vi "HFRR ADV v043.vi"() -> ()   [LabVIEW 2025] (continued)
  # "Calibration completed successfully. The measured stroke length is within the acceptable tolerance range of the factory calibration value."
  # "Calibration failed. The measured stroke length differs from the factory calibration value by more than 20%. Please perform the calibration again."
  # "Step 1 — Ball Holder"
  # "Remove the ball holder by loosening and removing the center screw for Friction calibration."
  # "Step 2 — Disc Holder"
  # "Remove the disc holder by loosening and removing the opposing screws. Clean any fluid present in the disc holder."
  # "Step 3 — Calibration Head"
  # "Place the calibration holder in position and securely tighten the center screw."
  # "Step 4 — Calibration Holder"
  # "Place the calibration holder in position and tighten the two securing screws"
  # "Step 5 — Tare (Spring at Free Length)"
  # "Ensure the spring is at its contact (compressed) length — the micrometer head is in contact. Click Tare Sensor to zero the friction force baseline."
  # "Step 6 — Measure Friction Force"
  # "Run the Actual Test to measure Friction Force."
  # "Calibration in Progress"
  # "Step 7 — CALIBRATION RESULT"
  # "Calibration completed successfully. The measured friction force is within the acceptable tolerance range of the factory calibration value."
  # "Calibration failed. The measured friction force differs from the factory calibration value . Please perform the calibration again."
  # "Spring Constant: k = 1.000 N/mm\nSpring force |F| = k Ч d"
  # "Calibrates the sample/bath temperature sensor. \nUsed for test specimen and lubricant temperature measurement."
  # "Calibrates the ambient air temperature sensor. \nUsed for environmental chamber monitoring."
  # "Set B\n60 °C\nHigh-point calibration"
  # "Set A\n0 °C\nIce-point calibration"
  # "Set B\n60 °C\nHigh-point calibration"
  # "Set A\n0 °C\nIce-point calibration"
  # "Select Temperature Sensor"
  # "Choose which temperature sensor you are calibrating. Both use the same two-\npoint procedure: 0 °C (ice-point) and 60 °C (high-point)."
  # "Step 1 — Reference Instrument Setup"
  # "Connect a calibrated reference to the DUT port. This calibration performs two sets: one at 0 °C and one at 60 °C."
  # "Set A\n0 °C\nIce-point calibration"
  # "Set B\n60 °C\nHigh-point calibration"
  # "Allow the temperature bath to stabilise for at least 2 minutes at each set-point before recording the reading."
  # "Step 2 — Set A:  0 °C Calibration"
  # "Connect the  0 °C reference connector. Wait for the temperature to stabilise. Once stable, and click Record Point."
  # "Step 3 — Set B:  60 °C Calibration"
  # "Connect the  60 °C reference connector. Wait for the temperature to stabilise. Once stable, and click Record Point."
  # "Sample Temperature Calibration Complete"
  # "Sample Temperature Calibration PASSED\nMax deviation 0.200 °C — within ±0.5 °C tolerance. Two-point correction applied (0 °C & 60 °C)."
  # "Sample  Temperature Calibration Failed\nmeasured Sample Temperature differs from the factory calibration value"
  # "Step 1 — Reference Instrument Setup"
  # "Connect a calibrated reference to the DUT port. This calibration performs two sets: one at 0 °C and one at 60 °C."
  # "Set A\n0 °C\nIce-point calibration"
  # "Set B\n60 °C\nHigh-point calibration"
  # "Allow the temperature bath to stabilise for at least 2 minutes at each set-point before recording the reading."
  # "Step 2 — Set A:  0 °C Calibration"
  # "Connect the  0 °C reference connector. Wait for the temperature to stabilise. Once stable, and click Record Point."
  # "Step 3 — Set B:  60 °C Calibration"
  # "Connect the  60 °C reference connector. Wait for the temperature to stabilise. Once stable, and click Record Point."
  # "Air Temperature Calibration Complete"
  # "Air Temperature Calibration PASSED\nMax deviation 0.200 °C — within ±0.5 °C tolerance. Two-point correction applied (0 °C & 60 °C)."
  # "Air  Temperature Calibration Failed\nmeasured Sample Temperature differs from the factory calibration value"
  # "System Control Commands\nS;1 - Starts the full automation cycle (Runs Priming-humidify till 70RH sequence first, then switches to Maintenance).\nS;0 - Stops the system immediately and enters Standby mode (Safe State: All actuators OFF).\nM;1 - Skips the priming sequence and jumps directly to Maintenance mode (PID control).\nR;1 - Resets the logic state machine and clears all errors, returning to Standby.\nService Mode (Manual Control)\nX;1 - Enters Manual Service Mode. This disables all automatic logic, sensor safety checks, and timers.\nX;0 - Exits Manual Service Mode and returns to Standby (Safe State).\nActuator Commands (Only work after sending X;1)\nP;[0-255] - Sets the Pump PWM. Note that this is Active Low (0 = Max Flow, 255 = Pump OFF).\nF;I;[0-255] - Sets the Intake Fan speed (0 = OFF, 255 = Max Speed).\nF;O;[0-255] - Sets the Exhaust Fan speed (0 = OFF, 255 = Max Speed).\nD;1 - Turns the Dehumidifier Relay ON.\nD;0 - Turns the Dehumidifier Relay OFF."
  # "%RH"
  # "ISO : WS1.4"
  # "Start test and end test log--- done\nDisable heater ON and Humidity ON during the test --- done\ntemprature and ---done\nhumidity reach log\nauto start run true logic and log\nmanual start log once"
  # "Reference Fluid Information"
  # "Note:\nMake sure to place all images in the folder \"C:\\WinDucom\\im\" before clicking on \"Import Image.\""
  # "NOTE:\nPlace all the images in the path \"C:\\WinDucom\\im\" before clicking on Import Image"
  # "Wear Scar Measurements"
  # "Reference Fluid Information"
  # "Graph :"
types:
  T1 = enum32{"Home", "Dashboard", "Imaging", "Report", "Analysis", "About", "Test Setup", "Advance", "Calibration"}
  T2 = enum32{"HOME", "Test Setup", "Acquire", "Adv Scar", "Adv Scar Report", "Compare Files", "Calibration", "About", "Advance", "Mooha"}
  T3 = enum16{"ASTM D6079", "ISO 12156", "CEC F-096-A-06", "Custom"}
  T4 = enum32{"Dashboard 1", "Dashboard 2", "Dashboard 3"}
  T5 = enum32{"COF", "Friction", "ECR", "Temperature", "Stroke"}
  T6 = enum32{"Coefficient Of Friction", "Air Temperature", "Humidity", "Stroke", "Sample Temperature", "Electrical Contact Resistance", "Frequency", "Air Temp vs Rh"}
  T7 = enum32{"Main", "Stroke", "Friction", "Temperature"}
  T8 = enum32{"Stroke Calibration", "Friction Force Calibration", "Temperature Calibration", "Default"}
  T9 = enum32{"Step 1", "Step 2", "Step 3", "Step 4", "Step 5", "Step 6", "Step 7", "Step 8", "Step 9"}
  T10 = enum32{"Test Progress", "Stroke Points Completed"}
  T11 = enum32{"Page 1", "Page 2", "Page 3", "Page 4", "Page 5", "Page 6"}
  T12 = enum32{"Main", "Step 1", "Step 2", "Step 3", "Step 4", "Air Step 1", "Air Step 2", "Air Step 3", "Air Step 4"}
  T13 = enum32{"Air Temperature", "Sample Temperature", "Default"}
  T14 = enum32{"COMMUNICATION", "CALIBRATION", "Temp Variables", "Camera", "WO 2465 (1)", "WO 2465 (2)", "WO 2465 (3)"}
  T15 = typedef "Auto Start enum.ctl" = enum16{"Init", "Humidity & Temperature On", "Reach point", "Maintain Stage", "Start Stage", "close", "Exit"}
  T16 = typedef "imagedata.ctl" = cluster{"image type":i32, "image depth":i32, "image":u8[], "mask":u8[], "colors":u32[], "Rectangle":cluster{"left":i16, "top":i16, "right":i16, "bottom":i16}}
  T17 = enum32{"HOME", "Test Setup", "Acquire", "Compare Files", "Print Report", "About", "Advance", "Mooha"}
  T18 = cluster{"Read Heave and Surge":string, "Bytes at Heave Port":dbl, "Heave and Surge COM Port:":refnum<visa-resource-name>, "Com Port 2":refnum<visa-resource-name>, "Residual Due":string, "Heave COM Status 2":bool, "Heave COM Status":bool, "Port 2":bool, "Sway PPR":dbl, "Surge PPR":dbl, "Heave PPR":dbl, "Sway Pitch":dbl, "Surge Pitch":dbl, "Heave Pitch":dbl, "Sway Pulses/mm":dbl, "Surge Pulses/mm":dbl, "Heave Pulses/mm":dbl, "inner loop":dbl, "Read Heave and Surge 2":string, "String 36":string, "Write S":bool, "WriteCC1":string[], "Heave COM Loop":i32, "LastCom":string, "EXIT":bool, "Error Heave":errorcluster}
  T19 = enum8{"Enabled", "Disabled", "Disabled and Grayed Out"}
  T20 = cluster{"Read Uno":string, "Bytes at Heave Port":dbl, "UNO COM Port:":refnum<visa-resource-name>, "UNO COM Port: 2":refnum<visa-resource-name>, "Residual Due":string, "UNO COM Status 2":bool, "UNO COM Status":bool, "Port 2":bool, "Sway PPR":dbl, "Surge PPR":dbl, "Heave PPR":dbl, "Sway Pitch":dbl, "Surge Pitch":dbl, "Heave Pitch":dbl, "Sway Pulses/mm":dbl, "Surge Pulses/mm":dbl, "Heave Pulses/mm":dbl, "inner loop":dbl, "Read Heave and Surge 2":string, "String 36":string, "Write S":bool, "WriteCC1":string[], "Heave COM Loop":i32, "LastCom":string, "EXIT":bool, "Error Heave":errorcluster}
  T21 = enum32{"HOME", "Test Setup", "Acquire", "Adv Scar", "Adv Scar Report", "Compare Files", "About", "Advance", "Mooha"}
  T22 = typedef "POST ANALYSIS ENUM.ctl" = enum16{"OPEN EXE", "INIT", "OPEN FILE", "FIT", "DRAW REC", "DRAW LINE", "PAN", "ZOOM IN", "ZOOM OUT", "SET ZOOM", "CLEAR ROI", "GET MEASUREMENTS", "RESIZE MODE", "STREAM START", "STREAM STOP", "SHOW UI", "MINIMIZE UI", "HIDE UI", "CKISE APP", "CLOSE CONNECTION", "SAVE IMAGE", "SET ROI COLOR", "READ", "TCP CHECK", "CLOSE"}
  T23 = typedef "CAMERA LIVE FEED ENUM.ctl" = enum16{"OPEN EXE", "INIT", "READ", "CAMERA CONNECT", "CAMERA START", "CAMERA STOP", "CAMERA GRAY", "CAMERA RGB", "CAMERA MINIMIZE", "CAMERA CLOSE", "CAMERA MODE LIST", "CAMERA MODE SET", "CAMERA RESTORE", "CAMERA SAVE", "CLOSE"}
  T24 = enum16{"Always On", "Always Off", "Off While Running"}
  T25 = enum32{"Home", "Dashboard", "Imaging", "Report", "Analysis", "About", "Test Setup", "Advance"}
  T26 = cluster{"File Name":string, "Test Method":string, "Operator":string, "Fuel Description":string, "Date and time":string}
  T27 = enum32{"Home", "Dashboard", "Imaging", "Report", "Analysis", "About", "Test Setup"}
  T28 = enum32{"HOME", "Test Setup", "Acquire", "Compare Files", "About", "Advance", "Mooha"}
  T29 = typedef "NI_ReportGenerationCore.lvlib/HTML Report Image Alignment.ctl" = enum16{"(default)", "LEFT", "RIGHT", "TOP", "TEXTTOP", "MIDDLE", "ABSMIDDLE", "BASELINE", "BOTTOM", "ABSBOTTOM"}
  T30 = cluster{"y":dbl, "LVDT STROKE DISPLAY":dbl, "y":dbl}
  T31 = enum16{"INIT", "READ", "MANUAL WRITE", "WRITE", "CLOSE", "ERROR INIT"}
diagram:
  w7 = 0.0 ("ch0_filt")
  w9 = -9999999.0 ("max_ch0")
  w10 = 9999999.0 ("min_ch0")
  w21 = FALSE ("Visible")
  w22 = T19."Enabled" ("Disabled")
  w25 = FALSE ("Visible")
  w24 = FALSE ("Humidity Off Command")
  w40 = "" ("USER ID")
  (unwired) T21."HOME" ("Main Tab")
  # "Temperature Continue Air Step 2"
  # "[CH1]    - FF\n[CH2]   - TEMPERATURE\n[CH3]    - Humidity\n[CH4]    - AIR TEMP\n[CH5]\\- Visa Uno\n[CH6] \\- Visa Due\n[CH7]  \\- file path\n[CH8]   - Displacement Gain\n[CHA]   - Stroke Gain\n[CHB]   - Stroke PID Gain\n[CHC]   -Language Selection\n[CHD]   -Power +\n[CHE]   -Power_\n[CHF]   -Heater\n[CHG]   -Humidity Wet\n[CHH]   -Humidity Dry\n[CHI]   -Integral Time \n[CHIJ   -Air intercept\n[CHI]   -Temp Intercept"
  n1 = local write "Cal Password"("" ("Cal Password")) -> ()
  n2 = property on="Auto Start Test" class="Bool (strict)"("Visible"=TRUE) -> ()  [unwired: 2 in, 2 out]
  n3 = property on="Friction Force Calibration Result Tab" class="TabCtl (strict)"("Visible"=FALSE) -> ()  [unwired: 2 in, 2 out]
  n4 = property on="FRICVALZ 2" class="Bool (strict)"("DisabledEnum"=w22) -> ()  [unwired: 2 in, 2 out]
  n5 = property on="FRICVALZ 4" class="Bool (strict)"("DisabledEnum"=w22) -> ()  [unwired: 2 in, 2 out]
  n6 = property on="FRICVALZ 3" class="Bool (strict)"("DisabledEnum"=w22) -> ()  [unwired: 2 in, 2 out]
  n7 = property on="About" class="Clust (strict)"("Visible"=FALSE) -> ()  [unwired: 2 in, 2 out]
  n8 = property on="Wrong Password" class="Str"("Visible"=w21) -> ()  [unwired: 2 in, 2 out]
  n9 = property on="Calibration 2" class="TabCtl (strict)"("Visible"=w21) -> ()  [unwired: 2 in, 2 out]
  n10 = local write "Temperature Selection"(T13."Default" ("Temperature Selection")) -> ()
  n11 = flat-sequence {
    tunnel: [w69] -> w6
    tunnel: [w114] -> w32
    tunnel: w6 -> [w109]
    tunnel: [w115] -> w34
    tunnel: w32 -> [w115]
    tunnel: w34 -> [w175]
    tunnel: [w175] -> w33
    tunnel: w33 -> [w206]
    tunnel: [w206] -> w43
    tunnel: w43 -> [w213]
    tunnel: [w219] -> w31
    tunnel: [w207] -> w30
    tunnel: [w261] -> w5
    tunnel: [w260] -> _
    tunnel: w31 -> [w260]
    tunnel: w30 -> [w261]
    frame #0 {
      n12 = call "CLOSE CONNECTION.vi"("error in (no error)"="error in (no error) 2") -> ("error out"=w74:errorcluster)  [unwired: 10 in]
      n13 = call <vilib>:"Clear Errors.vi"("error in (no error)"=w74) -> ("error out"=w73:errorcluster)  [unwired: 5 in, 1 out]
      n14 = disable-structure shown="Enabled" {
        disable-tunnel: w73 -> [w101 _]
        disable-tunnel: [w100 _] -> w72
        frame Enabled {
          n15 = call <userlib>:"Fit VI window to Largest Dec.vi"("error in (no error)"=w101, "border spacing (2 px)"=1) -> ("error out"=w104:errorcluster, "dup VI Ref"=w108:refnum<vi>)  [unwired: 4 in]
          n16 = invoke on="Invoke Node" class="VI" method="FP.Run-Time Position.Maximized"(reference=w108, error in=w104) -> (error out=w105:errorcluster)  [unwired: 2 in, 3 out]
          n17 = call <vilib>:"Clear Errors.vi"("error in (no error)"=w105) -> ("error out"=w107:errorcluster)  [unwired: 5 in, 1 out]
          n18 = control-ref of="This VI"() -> (w99:refnum<vi>)
          n19 = invoke on="Invoke Node" class="VI" method="Default Vals.Reinit All"(reference=w99, error in=w107) -> (reference out=w103:refnum<vi>, error out=w102:errorcluster)  [unwired: 1 in, 1 out]
          n20 = Close Reference(reference=w103, error in (no error)=w102) -> (error out=w100:errorcluster)
        }
        frame Disabled {
        }
      }
      n21 = call "Stall Data Flow.vim"("value in"=w72, "milliseconds to wait"=u32 2000) -> ("value out"=w71:errorcluster)  [unwired: 1 out]
      n22 = call "Read Config.vi"("error in (no error)"=w71) -> ("error out"=w69:errorcluster, "STROKE PARAMETERS"=w80:dbl[], "ADC PARAMETERS"=w81:dbl[], "PID  PARAMETERS"=w82:dbl[], "CALIBRATION PARAMETERS"=w67:string[], "Stroke Calibration"=w79:string)  [unwired: 5 in]
      n23 = Index Array(array=w80) -> (element #1=w97:dbl, element #2=w98:dbl)  [unwired: 2 in]
      n24 = Index Array(array=w67) -> (element #1=w66:string, element #2=w65:string, element #3=w64:string, element #4=w63:string, element #5=w62:string)  [unwired: 5 in]
      n25 = Index Array(array=w81) -> (element #1=w93:dbl, element #2=w94:dbl, element #3=w95:dbl, element #4=w96:dbl, element #5=w61:dbl)  [unwired: 5 in]
      n26 = Index Array(array=w82) -> (element #1=w84:dbl, element #2=w85:dbl, element #3=w86:dbl, element #4=w87:dbl, element #5=w88:dbl, element #6=w89:dbl, element #7=w90:dbl, element #8=w91:dbl, element #9=w92:dbl)  [unwired: 9 in]
      n27 = local write "STROKE FILTER"(w97) -> ()
      n28 = local write "Add up Stroke"(w98) -> ()
      n29 = local write "milliseconds to wait"(w84) -> ()
      n30 = local write "dt"(w85) -> ()
      n31 = local write "kp"(w86) -> ()
      n32 = local write "ki"(w87) -> ()
      n33 = local write "kd"(w88) -> ()
      n34 = local write "max_step_change"(w89) -> ()
      n35 = local write "max_amplitude"(w90) -> ()
      n36 = local write "min_amplitude"(w91) -> ()
      n37 = local write "startup_cmd"(w92) -> ()
      n38 = local write "VREF"(w93) -> ()
      n39 = local write "ADC_Resolution"(w94) -> ()
      n40 = local write "PIEZO_CAL_FACTOR"(w95) -> ()
      n41 = local write "NORMAL_FORCE"(w96) -> ()
      n42 = local write "Machine Serial Number"(w62) -> ()
      n43 = local write "STROKE CALIBRATION"(w66) -> ()
      n44 = local write "FRICTION CALIBRATION"(w65) -> ()
      n45 = local write "TEMPERATURE CALIBRATION"(w64) -> ()
      n46 = Fract/Exp String To Number(string=w63) -> (number=w68:dbl)  [unwired: 3 in, 1 out]
      n47 = local write "FF CAL EXCPTED VALUE"(w61) -> ()
      n48 = Spreadsheet String To Array(delimiter (Tab)=";", format string="", spreadsheet string=w79, array type (2D Dbl)=dbl[] []) -> (array=w83:dbl[])
      n49 = local write "Temperature diff"(w68) -> ()
      n50 = local write "calibration values"(w83) -> ()
    }
    frame #1 {
      n51 = property on="Auto Scar Check" class="Clust (strict)"("Visible"=TRUE) -> ()  [unwired: 2 in, 2 out]
      n52 = property on="Sign In" class="Bool (strict)"("DisabledEnum"=T19."Disabled" ("Disabled")) -> ()  [unwired: 2 in, 2 out]
      n53 = local write "sign in temp"(FALSE ("sign in temp")) -> ()
      n54 = call "dialog box.vi"("Status"="Before starting the test, verify that the microscope cable is connected.", "error in"=w109) -> ("error out"=w114:errorcluster)  [unwired: 8 in]
    }
    frame #2 {
      (unwired) TRUE ("Re-Initialise")
      # "kkkkk"
      # "C:\\Windows\\wndcm_pw_stdED hfrr.txt"
      # "C:\\LAB-IQ NXT"
      # "C:\\LAB-IQ NXT\\wndcm_pw_stdED hfrr.txt"
      # "password file"
      n55 = Current VI's Path() -> (path=w131:path)
      n56 = Strip Path(path=w131) -> (stripped path=w124:path)  [unwired: 1 out]
      n57 = local write "main tab sub"(enum32{"Page 1", "Page 2"}."Page 1" ("main tab sub")) -> ()
      n58 = local write "Main Tab Display"(T4."Dashboard 1" ("Main Tab Display")) -> ()
      n59 = local write "Main Tab"(T2."HOME" ("Main Tab")) -> ()
      n60 = Path To String(path=w124) -> (string=w126:string)
      n61 = Search/Split String(string=w126, search string/char (-)=".exe") -> (match + rest of string=w128:string)  [unwired: 1 in, 2 out]
      n62 = Match True/False String(2:".vi" ("false string"), 3:".exe" ("true string"), 4:w128) -> (0:w125:bool)  [unwired: 1 out]
      n63 = List Folder(path=path "C:/LAB-IQ" ("directory path"), pattern="*.txt") -> (filenames=w137:string[])  [unwired: 2 in, 3 out]
      n64 = case shown="True" w125 {
        tunnel: w124 -> [w146 w148]
        tunnel: [w146 w147] -> w122
        frame False {
        }
        frame True {
          n65 = Strip Path(path=w148) -> (stripped path=w147:path)  [unwired: 1 out]
        }
      }
      n66 = Search 1D Array(1D array=w137, element="wndcm_pw_stdED hfrr.txt") -> (index of element=w140:i32)  [unwired: 1 in]
      n67 = Equal?(x=w140, y=-1) -> (x = y?=w135:bool)
      n68 = Path To String(path=w122) -> (string=→"Gain path":string)
      n69 = case shown="True" w135 {
        frame False {
        }
        frame True {
          n70 = String To Byte Array(string="123\n") -> (unsigned byte array=w153:u8[])
          n71 = Array Size(array=w153) -> (size(s)=w152:i32)
          n72 = for {
            N: w152 -> [_]
            tunnel: w153 -> [w166]
            tunnel: [w163] -> w155 mode=indexing
            tunnel: w152 -> [w158]
            i -> [w156]
            n73 = Decrement(x=w158) -> (x-1=w159:i32)
            n74 = Index Array(array=w166, index=w156) -> (element=w165:u8)
            n75 = Equal?(x=w156, y=w159) -> (x = y?=w160:bool)
            n76 = Number To Decimal String(number=w165) -> (decimal integer string=w164:string)  [unwired: 1 in]
            n77 = Select(t="", s=w160, f="\r") -> (s? t:f=w157:string)
            n78 = Concatenate Strings(w164, w157) -> (w163:string)
          }
          n79 = local read "file path"() -> (w149:path)
          n80 = Concatenate Strings(w155) -> (w151:string)
          n81 = call <vilib>:"Write Characters To File.vi"("append to file? (new file:F)"=FALSE, "character string"=w151, "file path (dialog if empty)"=w149) -> ()  [unwired: 2 in, 1 out]
        }
      }
      n82 = local write "conststatus"(0.0 ("rpm value : 2")) -> ()
      n83 = local write "EVENT LOG"("") -> ()
      n84 = local write "COUNT"(0 ("COUNT")) -> ()
      n85 = local write "clk"(0.0 ("clk")) -> ()
      n86 = local write "Flag"(0.0 ("Flag")) -> ()
      n87 = local write "Lan flag"(0.0 ("Lan flag")) -> ()
      n88 = local write "Com flag"(u32 0 ("Com flag")) -> ()
      n89 = local write "refresh flag"(FALSE ("refresh flag")) -> ()
      "file path" <- path "C:/LAB-IQ/wndcm_pw_stdED hfrr.txt" ("file path")
      "FF buffer" <- dbl[] [] ("FF buffer")
    }
    frame #3 {
      # "C:\\WinDucom\\calibrate WO 2391.dcf"
      n90 = String To Path(string="C:\\LAB-IQ\\Image Calibrate v01.dcf") -> (path=w170:path)
      n91 = String To Path(string="C:\\LAB-IQ\\calibrate WO 2465.dcf") -> (path=w174:path)
      n92 = Open/Create/Replace File "Open File"(file path (use dialog)=w174) -> (refnum out=w173:refnum<file>)  [unwired: 5 in, 2 out]
      n93 = Open/Create/Replace File ("Open File")(file path (use dialog)=w170) -> (refnum out=w169:refnum<file>)  [unwired: 5 in, 2 out]
      n94 = for {
        N: 4 -> [_]
        tunnel: w169 -> [w181]
        i -> [w177]
        n95 = Read from Text File ("Read File")(file (use dialog)=w181) -> (text=w182:string)  [unwired: 3 in, 3 out]
        n96 = String Subset(string=w182, offset (0)=6, length (rest)=10 ("length (rest)")) -> (substring=w178:string)
        n97 = Fract/Exp String To Number(string=w178) -> (number=w176:dbl)  [unwired: 3 in, 1 out]
        n98 = case shown="3" w177 {
          tunnel: w176 -> [w183 w184 _ w185 _]
          frame 0 {
            n99 = local write "5x Gain"(w183) -> ()
          }
          frame 1 {
            n100 = local write "10x Gain"(w184) -> ()
          }
          frame 2 {
          }
          frame 3 {
            n101 = local write "100x gain"(w185) -> ()
          }
          frame 4, Default {
          }
        }
      }
      n102 = for {
        N: 24 -> [_]
        tunnel: w173 -> [w194]
        i -> [w188]
        (unwired) TRUE ("line mode (F)")
        n103 = Read from Text File "Read File"(file (use dialog)=w194) -> (text=w193:string)  [unwired: 3 in, 3 out]
        n104 = Match Pattern(string=w193, regular expression="]") -> (after substring=w191:string)  [unwired: 1 in, 3 out]
        n105 = String Subset(string=w193, offset (0)=5, length (rest)=10 ("length (rest)")) -> (substring=w186:string)
        n106 = Fract/Exp String To Number(string=w186) -> (number=w187:dbl)  [unwired: 3 in, 1 out]
        n107 = Match Pattern(string=w191, regular expression="-") -> (before substring=w189:string)  [unwired: 1 in, 3 out]
        n108 = case shown="18" w188 {
          tunnel: w187 -> [_ _ _ _ _ _ _ _ _ _ w201 _ _ _ _ _ _ _ _ _ _ _ _ _ _]
          tunnel: w189 -> [_ _ _ _ w197 w198 w199 _ _ _ _ _ _ _ _ _ _ _ _ _ w202 _ w203 w204 _]
          frame 0 {
          }
          frame 1 {
          }
          frame 2 {
          }
          frame 3 {
          }
          frame 4 {
            n109 = local write "Com Port 1"(w197) -> ()
          }
          frame 5 {
            n110 = local write "Com Port 2"(w198) -> ()
            n111 = local write "visa due"(w198) -> ()
          }
          frame 6 {
            n112 = String To Path(string=w199) -> (path=w200:path)
            n113 = local write "File Path"(w200) -> ()
          }
          frame 7 {
          }
          frame 8 {
          }
          frame 9 {
          }
          frame 10 {
            n114 = local write "Language Selection"(w201) -> ()
          }
          frame 11 {
          }
          frame 12 {
          }
          frame 13 {
          }
          frame 14 {
          }
          frame 15 {
          }
          frame 16 {
          }
          frame 17 {
          }
          frame 18 {
          }
          frame 21 {
          }
          frame 22 {
            n115 = local write "Com Port 3"(w202) -> ()
          }
          frame 23 {
          }
          frame 19 {
            n116 = local write "C3 :"(w203) -> ()
          }
          frame 20 {
            n117 = local write "Camera Port :"(w204) -> ()
          }
          frame 24, Default {
          }
        }
      }
    }
    frame #4 {
      n118 = Wait (ms)(milliseconds to wait=u32 1000) -> ()  [unwired: 1 out]
    }
    frame #5 {
      w222 = u32 2000 ("milliseconds to wait")
      w249 = u32 2000 ("milliseconds to wait")
      n119 = call "CAMERA LIVE FEED FGV.vi"("Enum - Menu"=CAMERA_LIVE_FEED_ENUM."OPEN EXE", "error in (no error)"=w213) -> ("error out"=w255:errorcluster)  [unwired: 8 in, 1 out]
      n120 = call "IMAGE ANALYSIS.vi"("Enum"=POST_ANALYSIS_ENUM."OPEN EXE", "error in"=w213) -> ("error out"=w210:errorcluster)  [unwired: 8 in, 1 out]
      n121 = call "Stall Data Flow.vim"("value in"=w255, "milliseconds to wait"=w249) -> ("value out"=w253:errorcluster)  [unwired: 1 out]
      n122 = call "Stall Data Flow.vim"("value in"=w210, "milliseconds to wait"=u32 8000) -> ("value out"=w209:errorcluster)  [unwired: 1 out]
      n123 = call "CAMERA LIVE FEED FGV.vi"("Enum - Menu"=CAMERA_LIVE_FEED_ENUM."INIT", "error in (no error)"=w253) -> ("error out"=w251:errorcluster)  [unwired: 8 in, 1 out]
      n124 = call "IMAGE ANALYSIS.vi"("Enum"=POST_ANALYSIS_ENUM."INIT", "error in"=w209) -> ("error out"=w207:errorcluster)  [unwired: 8 in, 1 out]
      n125 = case shown="Error .." w251 {
        selector: w251 -> [w256 _]
        tunnel: [w256 _] -> w250
        frame No Error {
        }
        frame Error {
          n126 = One Button Dialog(message="Camera initialization error.\nPlease Restart the software") -> ()  [unwired: 1 in, 1 out]
        }
      }
      n127 = property on="Camera Port :" class="CmbBox"() -> ("Strings[]"=w247:string[], "Value"=w248:string)  [unwired: 2 in, 2 out]
      n128 = Search 1D Array(1D array=w247, element=w248) -> (index of element=w246:i32)  [unwired: 1 in]
      n129 = Type Cast(type=30, x=w246) -> (*(type *) &x=w244:i32)
      n130 = call "Stall Data Flow.vim"("value in"=w250, "milliseconds to wait"=w249) -> ("value out"=w226:errorcluster)  [unwired: 1 out]
      n131 = Add(x=w244, y=48) -> (x+y=w225:i32)
      n132 = call "CAMERA LIVE FEED FGV.vi"("Enum - Menu"=CAMERA_LIVE_FEED_ENUM."CAMERA CONNECT", "error in (no error)"=w226, "CAMERA PORT"=w225) -> ("error out"=w235:errorcluster)  [unwired: 7 in, 1 out]
      n133 = call "Stall Data Flow.vim"("value in"=w235, "milliseconds to wait"=u32 5000) -> ("value out"=w236:errorcluster)  [unwired: 1 out]
      n134 = call "CAMERA LIVE FEED FGV.vi"("Enum - Menu"=CAMERA_LIVE_FEED_ENUM."CAMERA MODE LIST", "error in (no error)"=w236) -> ("error out"=w238:errorcluster)  [unwired: 8 in, 1 out]
      n135 = call "Stall Data Flow.vim"("value in"=w238, "milliseconds to wait"=w222) -> ("value out"=w237:errorcluster)  [unwired: 1 out]
      n136 = call "CAMERA LIVE FEED FGV.vi"("Enum - Menu"=CAMERA_LIVE_FEED_ENUM."READ", "error in (no error)"=w237) -> ("error out"=w224:errorcluster, "data out"=→"Camera List":string)  [unwired: 8 in]
      n137 = Type Cast(type=30, x=0) -> (*(type *) &x=w218:i32)
      n138 = call "Stall Data Flow.vim"("value in"=w224, "milliseconds to wait"=w222) -> ("value out"=w223:errorcluster)  [unwired: 1 out]
      n139 = Add(x=w218, y=48) -> (x+y=w216:i32)
      n140 = call "CAMERA LIVE FEED FGV.vi"("Enum - Menu"=CAMERA_LIVE_FEED_ENUM."CAMERA MODE SET", "error in (no error)"=w223, "CAMERA MODE"=w216) -> ("error out"=w220:errorcluster)  [unwired: 7 in, 1 out]
      n141 = call "Stall Data Flow.vim"("value in"=w220, "milliseconds to wait"=u32 2000) -> ("value out"=w240:errorcluster)  [unwired: 1 out]
      n142 = call "CAMERA LIVE FEED FGV.vi"("Enum - Menu"=CAMERA_LIVE_FEED_ENUM."CAMERA START", "error in (no error)"=w240) -> ("error out"=w241:errorcluster)  [unwired: 8 in, 1 out]
      n143 = call "Stall Data Flow.vim"("value in"=w241, "milliseconds to wait"=u32 1000) -> ("value out"=w242:errorcluster)  [unwired: 1 out]
      n144 = call "CAMERA LIVE FEED FGV.vi"("Enum - Menu"=CAMERA_LIVE_FEED_ENUM."CAMERA MINIMIZE", "error in (no error)"=w242) -> ("error out"=w219:errorcluster)  [unwired: 8 in, 1 out]
    }
    frame #6 {
      n145 = case shown="No Error" w260 {
        frame No Error {
          n146 = property on="Auto Scar Check" class="Clust (strict)"("Visible"=FALSE) -> ()  [unwired: 2 in, 2 out]
        }
        frame Error {
        }
      }
      n147 = property on="Sign In" class="Bool (strict)"("DisabledEnum"=T19."Enabled" ("Disabled")) -> ()  [unwired: 2 in, 2 out]
      n148 = local write "sign in temp"(TRUE ("sign in temp")) -> ()
    }
  }
  n149 = local write "Calibration Selection"(T8."Default" ("Calibration Selection")) -> ()
  n150 = local write "SCAR MEASURMENT"(enum32{"Auto Scar", "Manual Scar"}."Manual Scar" ("SCAR MEASURMENT")) -> ()
  n151 = local write "Temperature Off Command"(w24) -> ()
  n152 = local write "Main Dashboard Buttons"(T1."Home" ("Main Dashboard Buttons")) -> ()
  n153 = property on="Tab Control 6" class="TabCtl (strict)"("Visible"=FALSE) -> ()  [unwired: 2 in, 2 out]
  n154 = local write "Humidity Off Command"(w24) -> ()
  n155 = local write "CAMERA ROI MIN TEMP"(w24) -> ()
  n156 = local write "TEST FILE NAM,E SAVED"(w24) -> ()
  n157 = local write "LIVE FEED MIN TEMP"(w24) -> ()
  n158 = local write "SCAR MEASURMENT"(enum32{"Auto Scar", "Manual Scar"}."Manual Scar" ("SCAR MEASURMENT")) -> ()
  n159 = local write "Auto stop temp"(w25) -> ()
  n160 = local write "main tab sub"(enum32{"Page 1", "Page 2"}."Page 1" ("main tab sub")) -> ()
  n161 = while {
    stop <- w275 stop-if-true
    n162 = local read "Ambient Temperature"() -> (w273:dbl)
    n163 = local read "Sample Temperature 2"() -> (w272:dbl)
    n164 = Wait (ms)(milliseconds to wait=u32 200) -> ()  [unwired: 1 out]
    n165 = local write "Sensor value"(w273) -> ()
    n166 = local write "Sensor value"(w273) -> ()
    n167 = local write "Sensor value"(w272) -> ()
    n168 = local write "Sensor value"(w272) -> ()
    n169 = local write "Temperature — Live (Set A: 0 °C)"(w273) -> ()
    n170 = local write "Temperature — Live (Set A: 60 °C)"(w273) -> ()
    n171 = local write "Temperature — Live (Set A: 60 °C)"(w272) -> ()
    n172 = local write "Temperature — Live (Set A: 0 °C)"(w272) -> ()
    n173 = case shown="True" "Save Button" {
      selector: "Save Button" -> [_ w331]
      frame False {
      }
      frame True {
        n174 = Not(x=w331) -> (.not. x?=w330:bool)
        n175 = local read "Temperature diff"() -> (w327:dbl)
        n176 = local read "Machine Serial Number"() -> (w316:string)
        n177 = local read "milliseconds to wait"() -> (w363:u32)
        n178 = local write "Save Button"(w330) -> ()
        n179 = local read "max_step_change"() -> (w368:dbl)
        n180 = local read "FF CAL EXCPTED VALUE"() -> (w314:dbl)
        n181 = local read "max_amplitude"() -> (w369:dbl)
        n182 = local read "min_amplitude"() -> (w370:dbl)
        n183 = local read "PIEZO_CAL_FACTOR"() -> (w374:dbl)
        n184 = local read "startup_cmd"() -> (w371:dbl)
        n185 = local read "NORMAL_FORCE"() -> (w375:dbl)
        n186 = local read "ADC_Resolution"() -> (w373:dbl)
        n187 = local read "kp"() -> (w365:dbl)
        n188 = local read "kd"() -> (w367:dbl)
        n189 = local read "calibration values"() -> (w378:dbl[])
        n190 = local read "dt"() -> (w364:dbl)
        n191 = local read "ki"() -> (w366:dbl)
        n192 = local read "STROKE FILTER"() -> (w376:i32)
        n193 = local read "Add up Stroke"() -> (w377:dbl)
        n194 = Number To Fractional String(number=w327) -> (F-format string=w326:string)  [unwired: 3 in]
        n195 = local read "VREF"() -> (w372:dbl)
        n196 = Insert Into Array(array=dbl[] [], new element #1=w363, new element #2=w364, new element #3=w365, new element #4=w366, new element #5=w367, new element #6=w368, new element #7=w369, new element #8=w370, new element #9=w371) -> (w379:dbl[])  [unwired: 1 in]
        n197 = Insert Into Array(array=dbl[] [], new element #1=w372, new element #2=w373, new element #3=w374, new element #4=w375, new element #5=w314) -> (w380:dbl[])  [unwired: 1 in]
        n198 = Array To Spreadsheet String(delimiter (Tab)=";", array=w378, 3:"" ("format string")) -> (spreadsheet string=w382:string)
        n199 = Insert Into Array(array=dbl[] [], new element #1=w376, new element #2=w377) -> (w381:dbl[])  [unwired: 1 in]
        n200 = Insert Into Array(array=string[] [], new element #1="STROKE CALIBRATION", new element #2="FRICTION CALIBRATION", new element #3="TEMPERATURE CALIBRATION", new element #4=w326, new element #5=w316) -> (w328:string[])  [unwired: 1 in]
        n201 = call "Write Config.vi"("Stroke Calibration"=w382, "CALIBRATION PARAMETERS"=w328, "STROKE PARAMETERS"=w381, "ADC PARAMETERS"=w380, "PID  PARAMETERS"=w379) -> ("error out"=w361:errorcluster)  [unwired: 6 in]
        n202 = call "Stall Data Flow.vim"("value in"=w361, "milliseconds to wait"=u32 2000) -> ("value out"=w362:errorcluster)  [unwired: 1 out]
        n203 = call "Read Config.vi"("error in (no error)"=w362) -> ("STROKE PARAMETERS"=w359:dbl[], "ADC PARAMETERS"=w358:dbl[], "PID  PARAMETERS"=w357:dbl[], "CALIBRATION PARAMETERS"=w322:string[], "Stroke Calibration"=w360:string)  [unwired: 5 in, 1 out]
        n204 = Index Array(array=w357) -> (element #1=w355:dbl, element #2=w354:dbl, element #3=w353:dbl, element #4=w352:dbl, element #5=w351:dbl, element #6=w350:dbl, element #7=w349:dbl, element #8=w348:dbl, element #9=w347:dbl)  [unwired: 9 in]
        n205 = Index Array(array=w358) -> (element #1=w346:dbl, element #2=w345:dbl, element #3=w344:dbl, element #4=w343:dbl, element #5=w313:dbl)  [unwired: 5 in]
        n206 = Index Array(array=w359) -> (element #1=w342:dbl, element #2=w341:dbl)  [unwired: 3 in, 1 out]
        n207 = Index Array(array=w322) -> (element #1=w319:string, element #2=w318:string, element #3=w317:string, element #4=w321:string, element #5=w315:string)  [unwired: 5 in]
        n208 = Spreadsheet String To Array(delimiter (Tab)=";", format string="", spreadsheet string=w360, array type (2D Dbl)=dbl[] []) -> (array=w356:dbl[])
        n209 = local write "STROKE CALIBRATION"(w319) -> ()
        n210 = local write "FRICTION CALIBRATION"(w318) -> ()
        n211 = local write "TEMPERATURE CALIBRATION"(w317) -> ()
        n212 = Fract/Exp String To Number(string=w321) -> (number=w320:dbl)  [unwired: 3 in, 1 out]
        n213 = local write "Machine Serial Number"(w315) -> ()
        n214 = local write "STROKE FILTER"(w342) -> ()
        n215 = local write "Add up Stroke"(w341) -> ()
        n216 = local write "VREF"(w346) -> ()
        n217 = local write "ADC_Resolution"(w345) -> ()
        n218 = local write "PIEZO_CAL_FACTOR"(w344) -> ()
        n219 = local write "NORMAL_FORCE"(w343) -> ()
        n220 = local write "FF CAL EXCPTED VALUE"(w313) -> ()
        n221 = local write "calibration values"(w356) -> ()
        n222 = local write "milliseconds to wait"(w355) -> ()
        n223 = local write "dt"(w354) -> ()
        n224 = local write "kp"(w353) -> ()
        n225 = local write "ki"(w352) -> ()
        n226 = local write "kd"(w351) -> ()
        n227 = local write "max_step_change"(w350) -> ()
        n228 = local write "max_amplitude"(w349) -> ()
        n229 = local write "min_amplitude"(w348) -> ()
        n230 = local write "startup_cmd"(w347) -> ()
        n231 = local write "Temperature diff"(w320) -> ()
      }
    }
    n232 = local read "USER ID"() -> (w270:string)
    n233 = local read "run test Calibration"() -> (w268:bool)
    n234 = disable-structure shown="Enabled" {
      disable-tunnel: [w282 w293] -> w269
      frame Disabled {
        n235 = local read "Point 1 - 0.2 mm"() -> (w292:bool)
        n236 = local read "Point 2 - 0.4 mm"() -> (w291:bool)
        n237 = local read "Point 3 - 0.6 mm"() -> (w290:bool)
        n238 = local read "Point 4 - 0.8 mm"() -> (w289:bool)
        n239 = local read "Point 5 - 1.0 mm"() -> (w288:bool)
        n240 = local read "Point 6 - 1.2 mm"() -> (w287:bool)
        n241 = And(x=w292, y=w291) -> (x .and. y?=w286:bool)
        n242 = And(x=w290, y=w289) -> (x .and. y?=w285:bool)
        n243 = And(x=w288, y=w287) -> (x .and. y?=w283:bool)
        n244 = And(x=w286, y=w285) -> (x .and. y?=w284:bool)
        n245 = And(x=w284, y=w283) -> (x .and. y?=w282:bool)
      }
      frame Enabled {
        n246 = local read "Point 5 - 1.0 mm"() -> (w293:bool)
      }
    }
    n247 = local read "START TEMP"() -> (w267:bool)
    n248 = local write "tested by 2"(w270) -> ()
    n249 = And(x=w267, y=w268) -> (x .and. y?=w266:bool)
    n250 = case shown="True" w266 {
      frame False {
        w294 = TRUE ("PAUSE")
        n251 = call "ELAPSED TIMER VI - Calibration.vi"("RESET"=w294, "PAUSE"=w294) -> ()  [unwired: 7 in, 3 out]
      }
      frame True {
        w297 = FALSE ("PAUSE")
        n252 = call "ELAPSED TIMER VI - Calibration.vi"("TARGET"=60.0, "RESET"=w297, "PAUSE"=w297) -> ("ELAPSED INDICATION"=w295:bool)  [unwired: 6 in, 2 out]
        n253 = case shown="False" w295 {
          frame False {
            n254 = local write "Friction Force Calibration Result Tab"(enum32{"Calibration Results", "Page 2"}."Calibration Results" ("Friction Force Calibration Result Tab")) -> ()
            n255 = property on="Friction Force Calibration Result Tab" class="TabCtl (strict)"("Visible"=FALSE) -> ()  [unwired: 2 in, 2 out]
          }
          frame True {
            n256 = stacked-sequence {
              frame #0 {
                n257 = local read "Friction"() -> (→"Friction cal":dbl)
                n258 = local write "run test Calibration"(FALSE ("run test Calibration")) -> ()
                n259 = local write "START TEMP"(FALSE ("START TEMP")) -> ()
              }
              frame #1 {
                n260 = Wait (ms)(milliseconds to wait=u32 1500) -> ()  [unwired: 1 out]
              }
              frame #2 {
                n261 = local write "Due Write"("VC;0") -> ()
              }
              frame #3 {
                n262 = Wait (ms)(milliseconds to wait=u32 1500) -> ()  [unwired: 1 out]
              }
              frame #4 {
                n263 = local write "Due Write"("VC;0") -> ()
              }
              frame #5 {
                n264 = property on="Friction Force Calibration Result Tab" class="TabCtl (strict)"("Visible"=TRUE) -> ()  [unwired: 2 in, 2 out]
                n265 = property on="Tab Control 6" class="TabCtl (strict)"("Visible"=FALSE) -> ()  [unwired: 2 in, 2 out]
              }
            }
          }
        }
      }
    }
    n266 = local read "Friction cal"() -> (w265:dbl)
    n267 = case shown="False" w269 {
      frame False {
        n268 = property on="Accept & Save" class="Bool (strict)"("DisabledEnum"=T19."Disabled" ("Disabled")) -> ()  [unwired: 2 in, 2 out]
        n269 = property on="Tab Control 5" class="TabCtl (strict)"("Value"=enum32{"OK", "NG"}."NG" ("Tab Control 5")) -> ()  [unwired: 2 in, 2 out]
      }
      frame True {
        n270 = property on="Accept & Save" class="Bool (strict)"("DisabledEnum"=T19."Enabled" ("Disabled")) -> ()  [unwired: 2 in, 2 out]
        n271 = property on="Tab Control 5" class="TabCtl (strict)"("Value"=enum32{"OK", "NG"}."OK" ("Tab Control 5")) -> ()  [unwired: 2 in, 2 out]
      }
    }
    n272 = Greater Or Equal?(x=w265, y="FF CAL EXCPTED VALUE") -> (x >= y?=w263:bool)
    n273 = case shown="False" w263 {
      selector: w263 -> [w276 w279]
      frame False {
        n274 = local write "FF PASS"(w276) -> ()
        n275 = local write "Friction Force result Tab"(enum32{"OK", "NG"}."NG" ("Friction Force result Tab")) -> ()
        n276 = property on="Accept & Save FF" class="Bool (strict)"("DisabledEnum"=T19."Disabled" ("Disabled")) -> ()  [unwired: 2 in, 2 out]
      }
      frame True {
        n277 = local write "Friction Force result Tab"(enum32{"OK", "NG"}."OK" ("Friction Force result Tab")) -> ()
        n278 = property on="Accept & Save FF" class="Bool (strict)"("DisabledEnum"=T19."Enabled" ("Disabled")) -> ()  [unwired: 2 in, 2 out]
        "FF PASS" <- w279
      }
    }
    n279 = local read "Quit"() -> (w275:bool)
  }
  n280 = local write "USERNAME"(w40) -> ()
  n281 = local write "Main Tab"(T2."HOME" ("Main Tab")) -> ()
  n282 = local write "USER ID"(w40) -> ()
  n283 = property on="Auto Scar Check  2" class="Clust (strict)"("Visible"=w25) -> (error out=w28:errorcluster)  [unwired: 2 in, 1 out]
  n284 = property on="Quit" class="Bool (strict)"("Value"=FALSE ("Quit")) -> (error out=w42:errorcluster)  [unwired: 2 in, 1 out]
  n285 = while {
    stop <- w383 stop-if-true
    n286 = event shown="[51] \"FF CONTINUE 5\": Value Change" {
      selector: _ -> [_ _ _ _ _ _ _ _ _ _ _ _ _ _ _ _ _ _ _ _ _ _ _ _ _ _ _ _ _ _ _ _ _ _ _ _ _ _ _ _ _ _ _ _ _ _ _ _ _ _ _ _ _ _ _ _ _]
      dyn-events: _ -> [_ _ _ _ _ _ _ _ _ _ _ _ _ _ _ _ _ _ _ _ _ _ _ _ _ _ _ _ _ _ _ _ _ _ _ _ _ _ _ _ _ _ _ _ _ _ _ _ _ _ _ _ _ _ _ _ _]
      timeout: 100 -> [_ _ _ _ _ _ _ _ _ _ _ _ _ _ _ _ _ _ _ _ _ _ _ _ _ _ _ _ _ _ _ _ _ _ _ _ _ _ _ _ _ _ _ _ _ _ _ _ _ _ _ _ _ _ _ _ _]